vi "TLB Native Dynamic Events ver 0.26c.vi"() -> ()   [LabVIEW 2018] (continued)
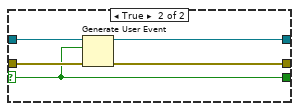
[diagram p2: hidden frame]
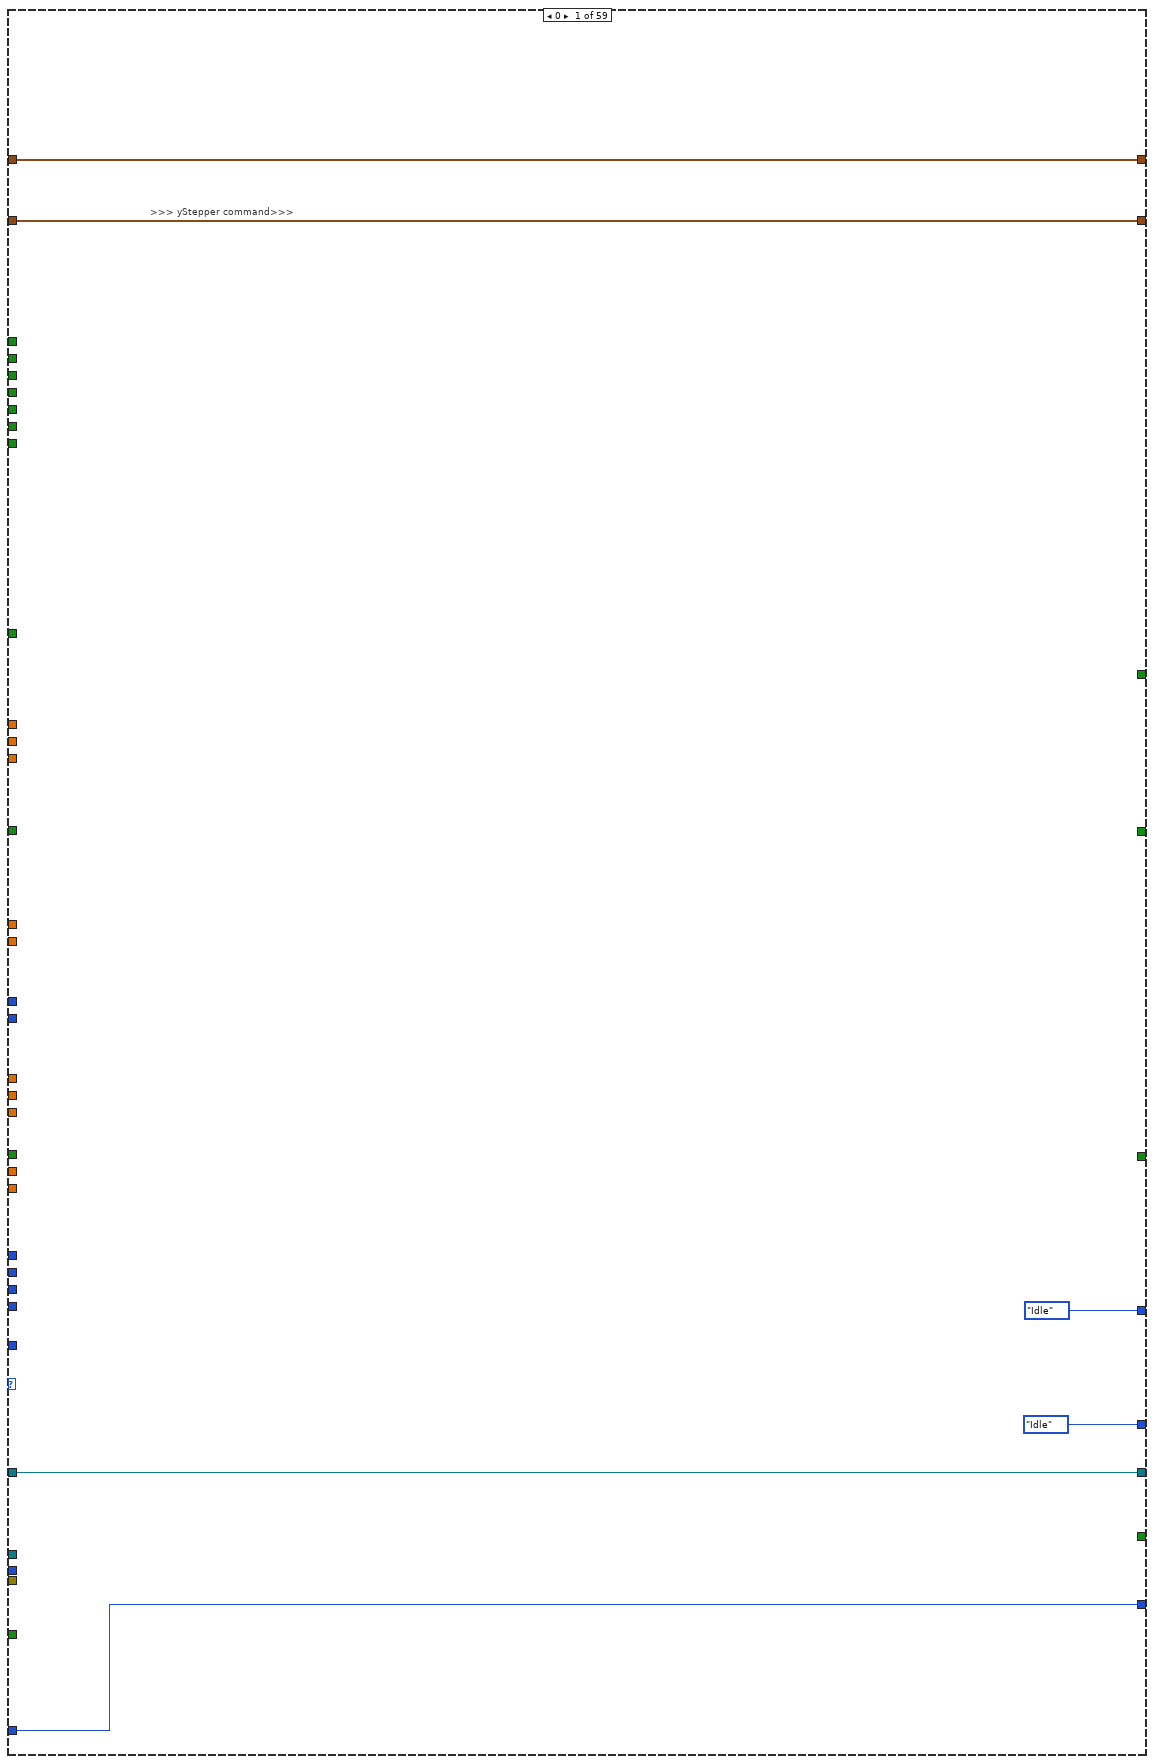
[diagram p5: hidden frame]
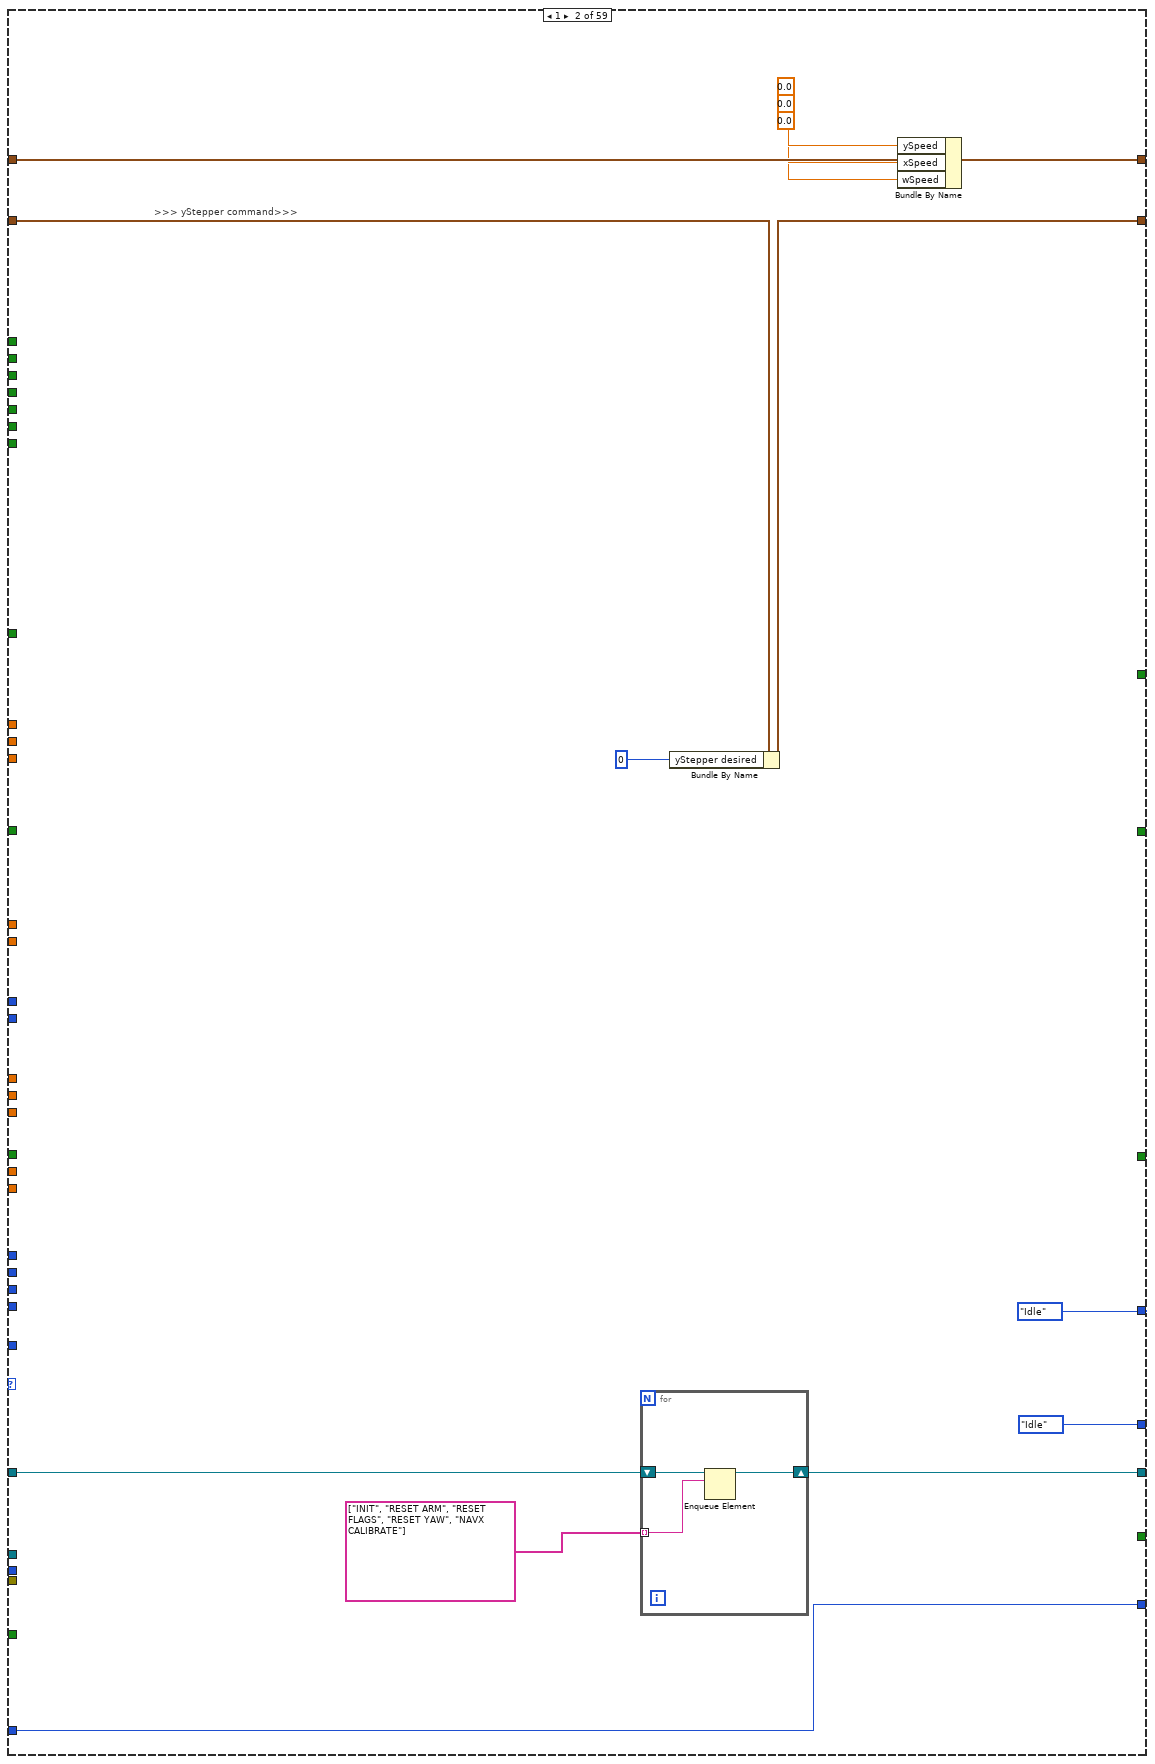
[diagram p6: hidden frame]
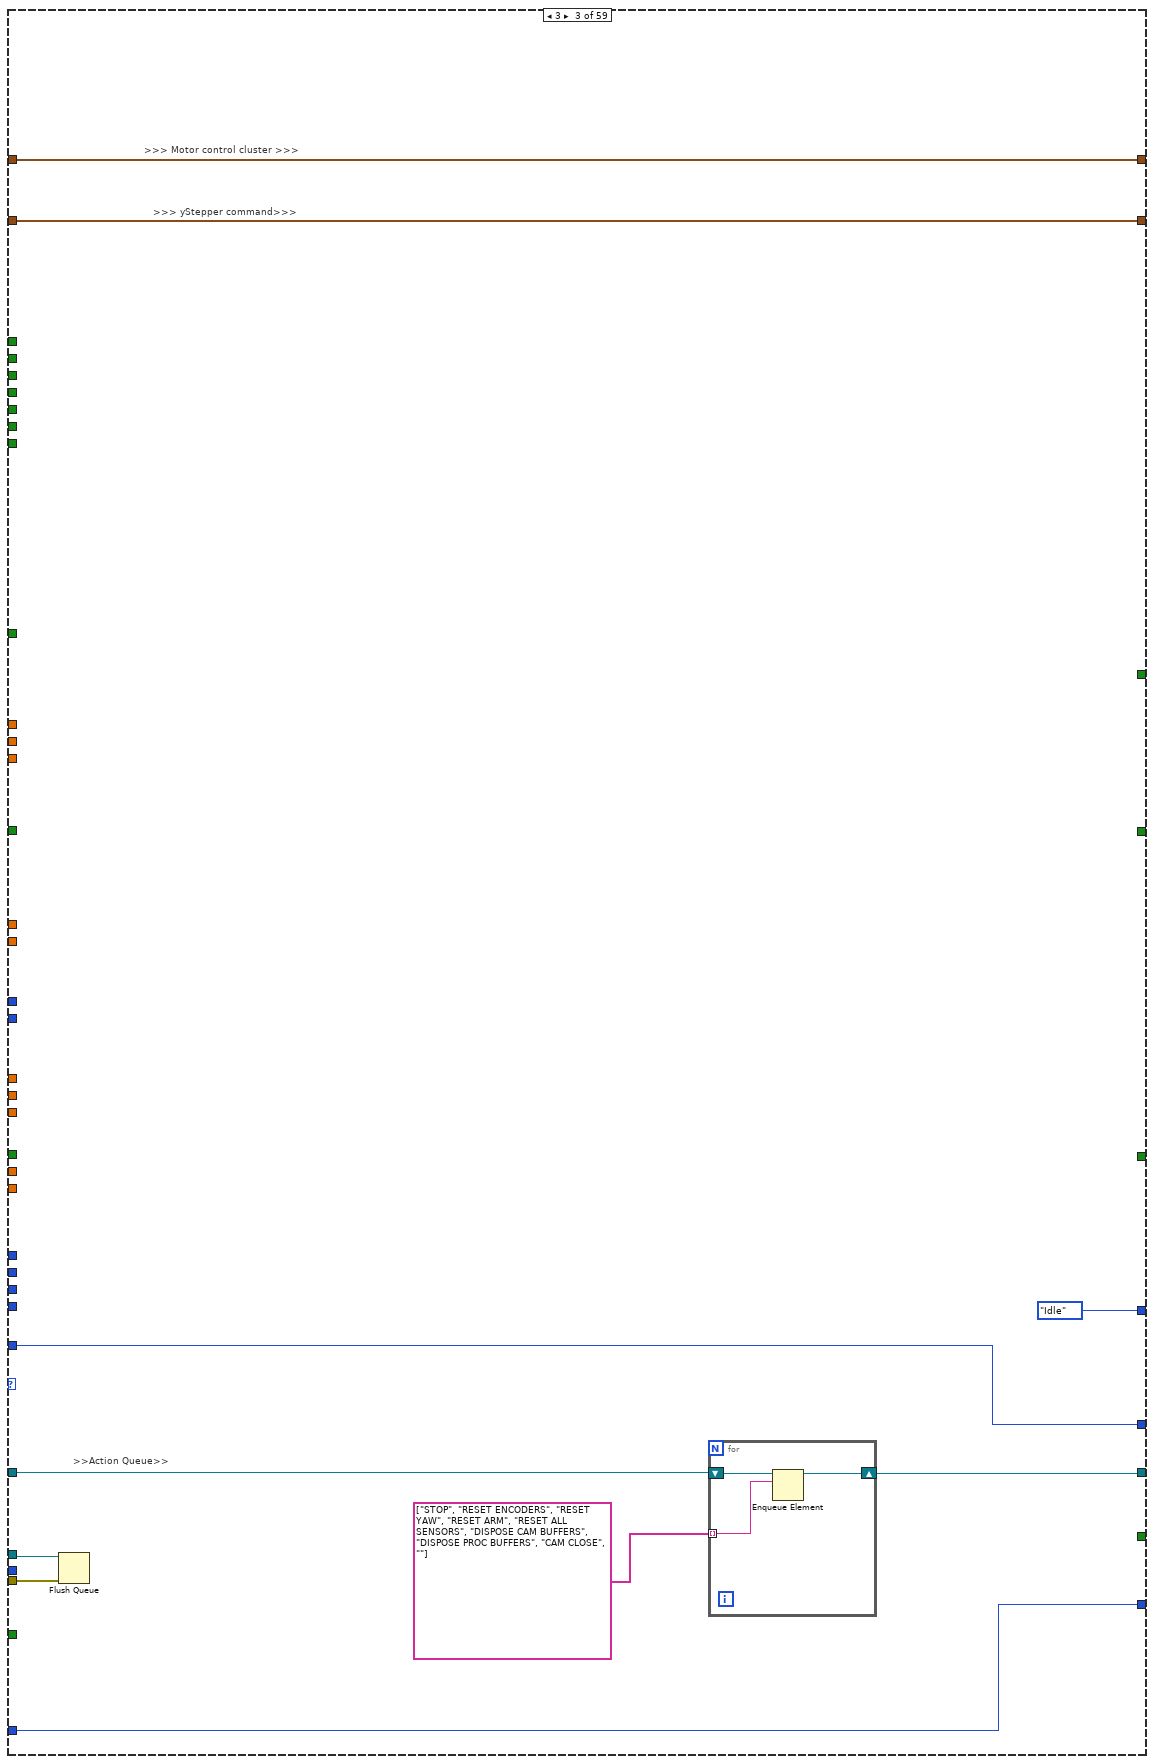
[diagram p7: hidden frame]
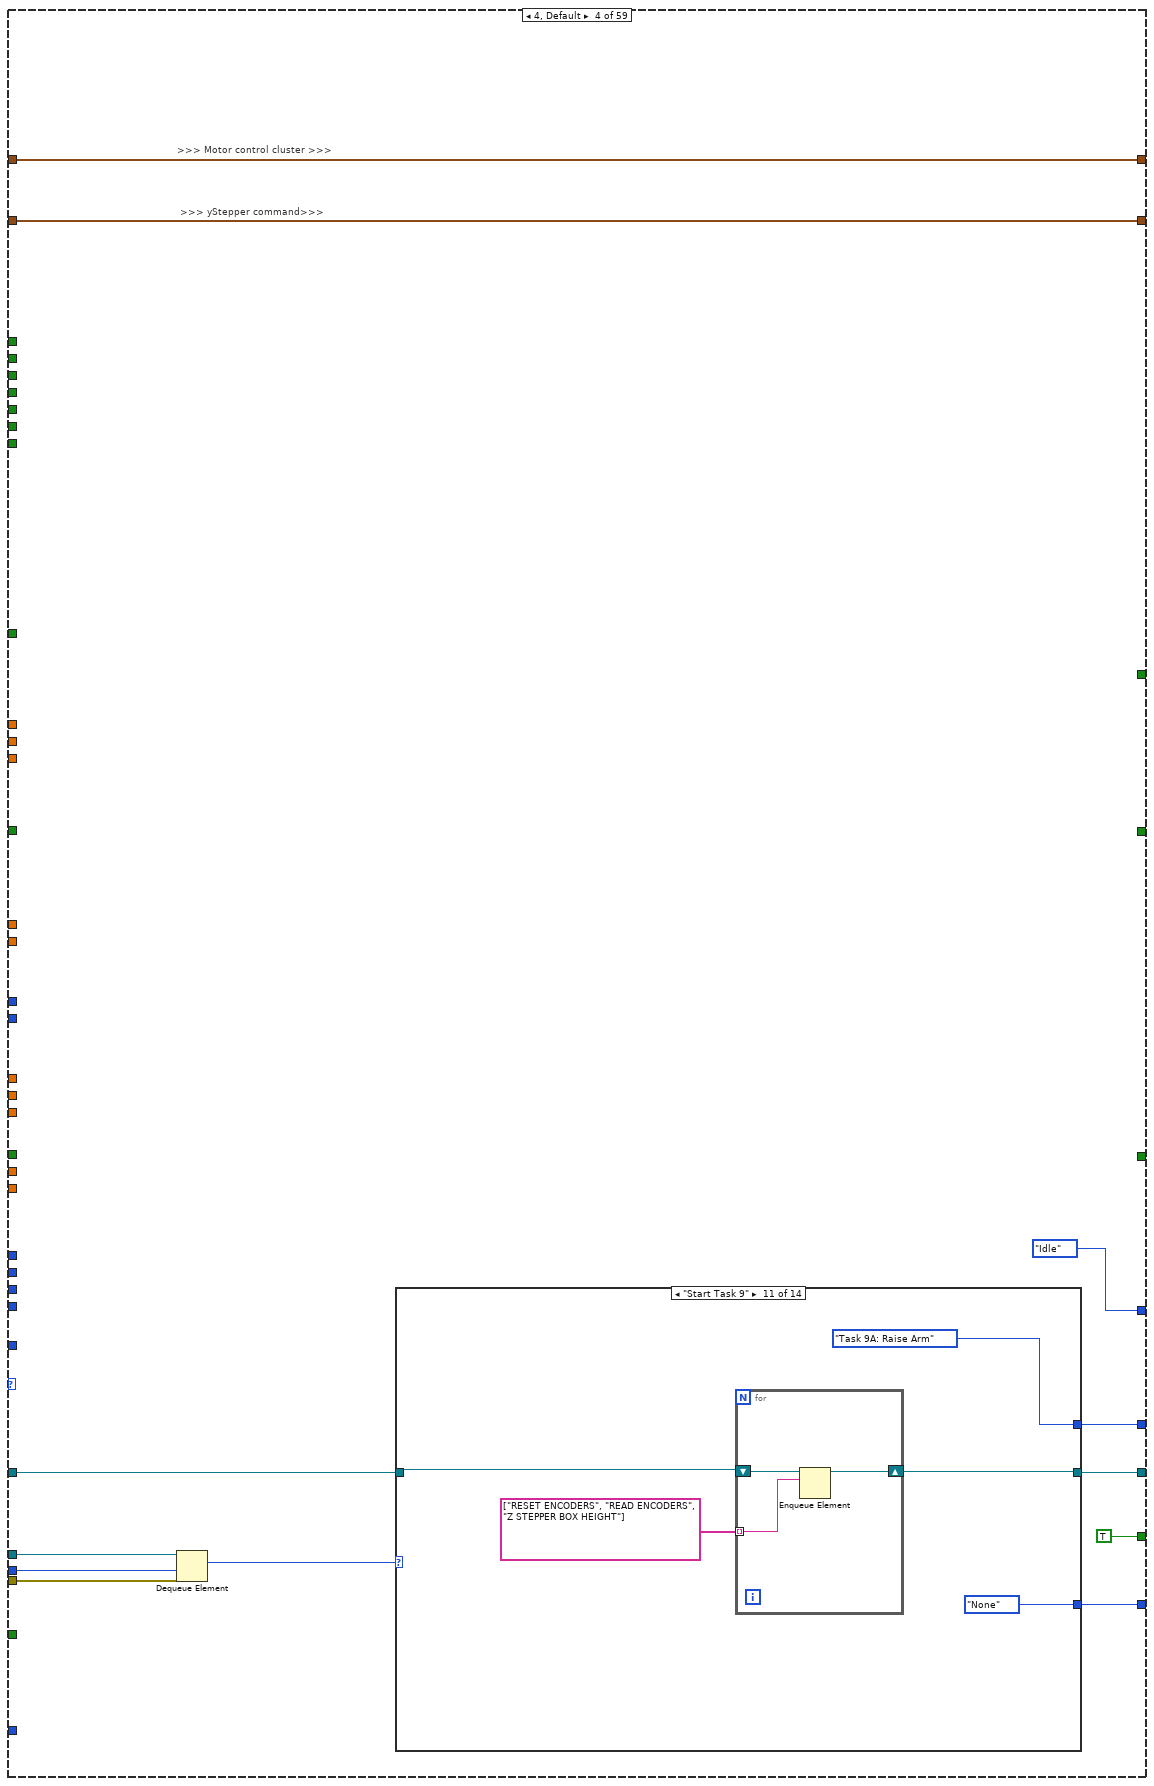
[diagram p8: hidden frame]
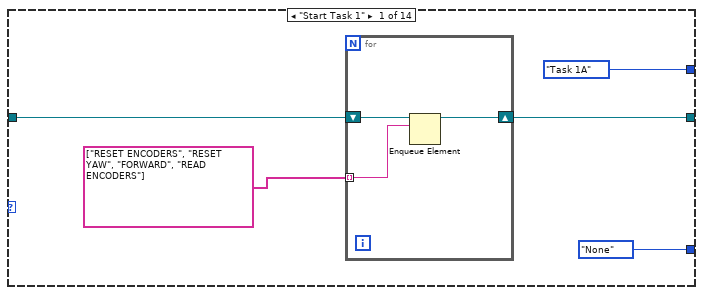
[diagram p9: hidden frame]
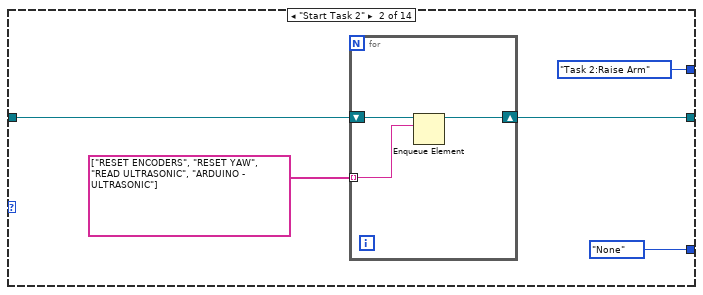
[diagram p10: hidden frame]
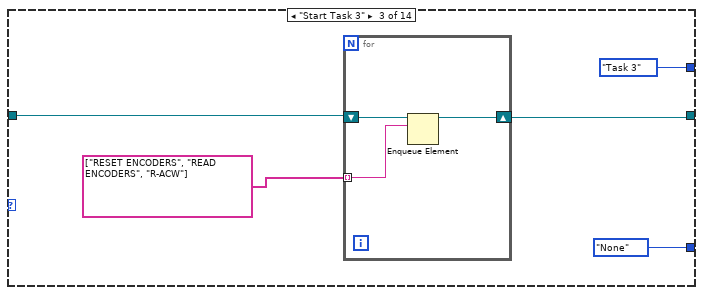
[diagram p11: hidden frame]
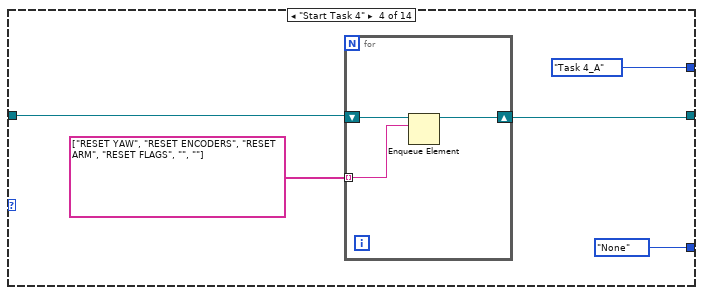
[diagram p12: hidden frame]
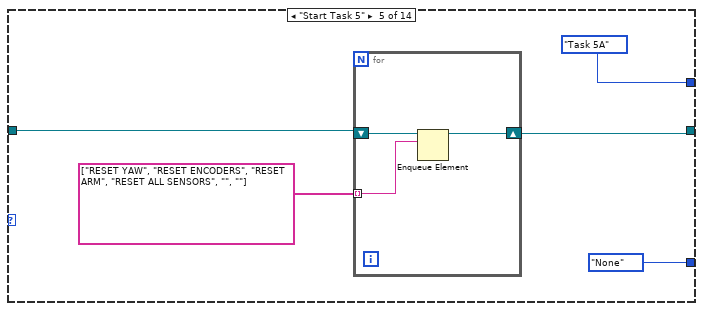
[diagram p13: hidden frame]
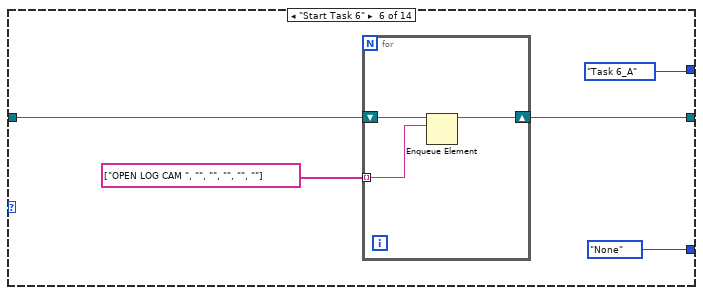
[diagram p14: hidden frame]
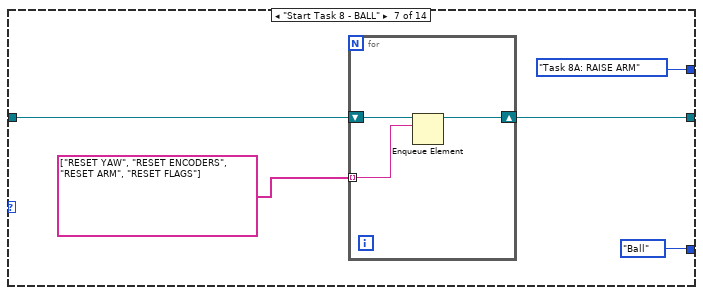
[diagram p15: hidden frame]
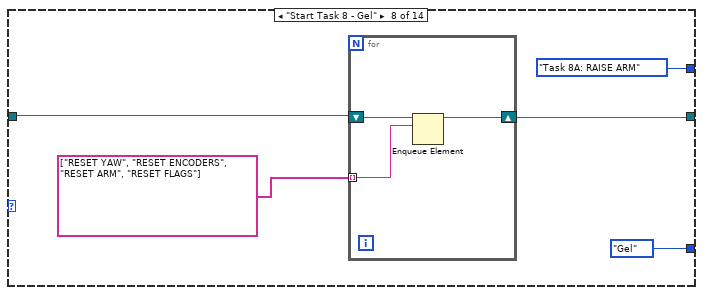
[diagram p16: hidden frame]
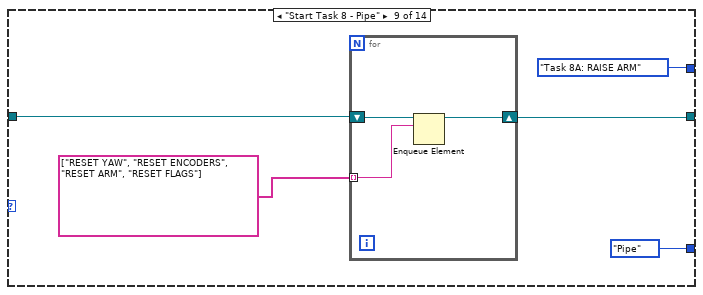
[diagram p17: hidden frame]
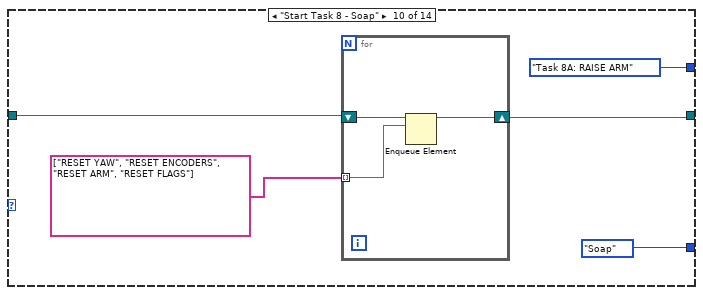
[diagram p18: hidden frame]
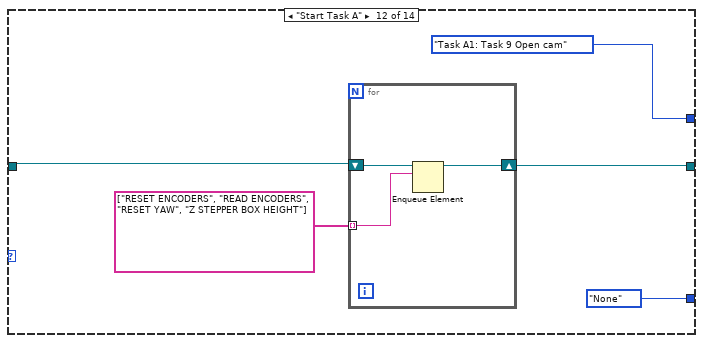
[diagram p19: hidden frame]
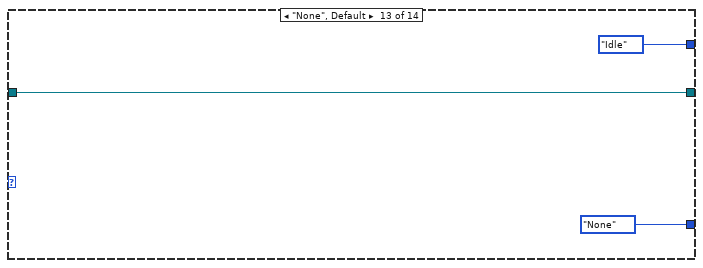
[diagram p20: hidden frame]
                  frame True {
                    n866 = for {
                      shift-right: [w2677] -> w2674
                      shift-left: w2675 -> [w2678]
                      tunnel: string[] ["STOP", "RESET ENCODERS", "RESET YAW", "OPEN LIFE CAM", "SET TIMER 2", "RESET FLAGS"] -> [w2676] mode=indexing
                      n867 = Enqueue Element(queue=w2678, element=w2676) -> (queue out=w2677:refnum<queue>)  [unwired: 2 in, 2 out]
                    }
                  }
                }
                n868 = Or(x=w2658, y=w2657) -> (x .or. y?=w2656:bool)
                n869 = Select(t=State_Type_Definitions,_for_0.26g_versions_and_later_2."True Stop" ("Enum"), s=w2657, f=State_Type_Definitions,_for_0.26d_versions_and_later."Task 9Q: SCAN IMAGE" ("Enum")) -> (s? t:f=w2659:u16)
                n870 = Select(t=w2659, s=w2656, f=State_Type_Definitions,_for_0.26d_versions_and_later."Task 9P: MOVE RIGHT" ("Enum")) -> (s? t:f=w2665:u16)
              }
              frame "Exit" {
                n871 = for {
                  shift-right: [w2685] -> w2682
                  shift-left: w2681 -> [w2686]
                  tunnel: string[] ["STOP", "RESET ENCODERS", "RESET YAW", "ARDUINO MODE 0"] -> [w2684] mode=indexing
                  n872 = Enqueue Element(queue=w2686, element=w2684) -> (queue out=w2685:refnum<queue>)  [unwired: 2 in, 2 out]
                }
              }
            }
          }
          frame 54 {
            # ">> Manual override >>"
            n873 = Dequeue Element(queue=w2695, timeout in ms (-1)=w2694, error in (no error)=w2693) -> (element=w2696:T10)  [unwired: 3 out]
            n874 = case shown="\"Start Task 1\", Default" w2696 {
              tunnel: [w2710 State_Type_Definitions,_for_0.26g_versions_and_later_2."True Stop" ("Enum")] -> w2688
              tunnel: [w2708 w2726] -> w2687
              tunnel: w2691 -> [w2707 w2723]
              tunnel: w2692 -> [w2701 _]
              tunnel: [State_Type_Definitions,_for_0.26g_versions_and_later_2."Idle" ("Enum") State_Type_Definitions,_for_0.26g_versions_and_later_2."Shutdown" ("Enum")] -> w2689
              tunnel: w2690 -> [w2700 _]
              frame "Start Task 1", Default {
                # ">> WIill proceed to part ii if not manual override >>"
                # ">>If ENABLE or Trigger is set to true>>"
                n875 = Or(x=w2700, y=w2701) -> (x .or. y?=w2702:bool)
                n876 = case shown="False" w2700 {
                  tunnel: [w2713 w2719] -> w2708
                  tunnel: w2707 -> [w2712 w2718]
                  frame False {
                    n877 = for {
                      shift-right: [w2715] -> w2713
                      shift-left: w2712 -> [w2716]
                      tunnel: string[] ["CAM ACQ", "START TIMER"] ("element") -> [w2714] mode=indexing
                      n878 = Enqueue Element(queue=w2716, element=w2714) -> (queue out=w2715:refnum<queue>)  [unwired: 2 in, 2 out]
                    }
                  }
                  frame True {
                    n879 = for {
                      shift-right: [w2721] -> w2719
                      shift-left: w2718 -> [w2722]
                      tunnel: string[] ["CLOSE CAM", "SET TIMER 5", "", "", "", ""] -> [w2720] mode=indexing
                      n880 = Enqueue Element(queue=w2722, element=w2720) -> (queue out=w2721:refnum<queue>)  [unwired: 2 in, 2 out]
                    }
                  }
                }
                n881 = Select(t=State_Type_Definitions,_for_0.26g_versions_and_later_2."True Stop" ("Enum"), s=w2701, f=State_Type_Definitions,_for_0.26g_versions_and_later_2."Task 9R: PROCESS COLOUR" ("Enum")) -> (s? t:f=w2704:T18)
                n882 = Select(t=w2704, s=w2702, f=State_Type_Definitions,_for_0.26d_versions_and_later."Task 9Q: SCAN IMAGE" ("Enum")) -> (s? t:f=w2710:u16)
              }
              frame "Exit" {
                n883 = for {
                  shift-right: [w2729] -> w2726
                  shift-left: w2723 -> [w2730]
                  tunnel: string[] ["STOP", "RESET ENCODERS", "RESET YAW", ""] -> [w2728] mode=indexing
                  n884 = Enqueue Element(queue=w2730, element=w2728) -> (queue out=w2729:refnum<queue>)  [unwired: 2 in, 2 out]
                }
              }
            }
          }
          frame 55 {
            # ">> Item Selection Bias >>"
            # ">>> Motor control cluster >>>"
            # ">>> yStepper command>>>"
            n885 = Dequeue Element(queue=w2736, timeout in ms (-1)=w2737, error in (no error)=w2738) -> (element=w2740:T10)  [unwired: 3 out]
            n886 = case shown="\"Start Task 1\", Default" w2740 {
              tunnel: w2734 -> [w2746 _]
              tunnel: [w2753 State_Type_Definitions,_for_0.26g_versions_and_later_2."True Stop" ("Enum")] -> w2732
              tunnel: w2739 -> [w2745 _]
              tunnel: w2735 -> [w2752 w2769]
              tunnel: [w2751 w2770] -> w2731
              tunnel: [State_Type_Definitions,_for_0.26g_versions_and_later_2."Idle" ("Enum") State_Type_Definitions,_for_0.26g_versions_and_later_2."Shutdown" ("Enum")] -> w2733
              frame "Start Task 1", Default {
                n887 = case shown="False" w2746 {
                  tunnel: w2752 -> [w2756 w2763]
                  tunnel: [w2757 w2762] -> w2751
                  frame False {
                    n888 = for {
                      tunnel: string[] ["START TIMER", "COLOUR PROCESSING", ""] ("element") -> [w2758] mode=indexing
                      shift-right: [w2760] -> w2757
                      shift-left: w2756 -> [w2759]
                      n889 = Enqueue Element(queue=w2759, element=w2758) -> (queue out=w2760:refnum<queue>)  [unwired: 2 in, 2 out]
                    }
                  }
                  frame True {
                    n890 = for {
                      shift-right: [w2765] -> w2762
                      shift-left: w2763 -> [w2766]
                      tunnel: string[] ["CLOSE CAM", "DISPOSE BUFFERS", "RESET ENCODERS", "RESET YAW", "RESET FLAGS", ""] -> [w2764] mode=indexing
                      n891 = Enqueue Element(queue=w2766, element=w2764) -> (queue out=w2765:refnum<queue>)  [unwired: 2 in, 2 out]
                    }
                  }
                }
                n892 = Or(x=w2746, y=w2745) -> (x .or. y?=w2744:bool)
                n893 = Select(t=State_Type_Definitions,_for_0.26g_versions_and_later_2."True Stop" ("Enum"), s=w2745, f=State_Type_Definitions,_for_0.26g_versions_and_later_2."True Stop" ("Enum")) -> (s? t:f=w2747:T18)
                n894 = Select(t=w2747, s=w2744, f=State_Type_Definitions,_for_0.26g_versions_and_later_2."Task 9R: PROCESS COLOUR" ("Enum")) -> (s? t:f=w2753:T18)
              }
              frame "Exit" {
                n895 = for {
                  shift-right: [w2773] -> w2770
                  shift-left: w2769 -> [w2774]
                  tunnel: string[] ["STOP", "RESET ENCODERS", "RESET YAW", "ARDUINO MODE 0"] -> [w2772] mode=indexing
                  n896 = Enqueue Element(queue=w2774, element=w2772) -> (queue out=w2773:refnum<queue>)  [unwired: 2 in, 2 out]
                }
              }
            }
          }
          frame 56 {
            # ">>> Motor control cluster >>>"
            # ">>> yStepper command>>>"
            # ">> Manual override >>"
            n897 = Dequeue Element(queue=w2786, timeout in ms (-1)=w2782, error in (no error)=w2785) -> (element=w2787:T10)  [unwired: 3 out]
            n898 = case shown="\"Start Task 1\", Default" w2787 {
              tunnel: [w2798 State_Type_Definitions,_for_0.26g_versions_and_later_2."True Stop" ("Enum")] -> w2780
              tunnel: [w2796 w2813] -> w2779
              tunnel: w2783 -> [w2795 _]
              tunnel: w2784 -> [w2789 _]
              tunnel: [State_Type_Definitions,_for_0.26g_versions_and_later_2."Idle" ("Enum") State_Type_Definitions,_for_0.26g_versions_and_later_2."Shutdown" ("Enum")] -> w2781
              tunnel: w2775 -> [w2788 _]
              frame "Start Task 1", Default {
                # ">> WIill proceed to part ii if not manual override >>"
                # ">>If ENABLE or Trigger is set to true>>"
                n899 = Or(x=w2788, y=w2789) -> (x .or. y?=w2790:bool)
                n900 = case shown="False" w2788 {
                  tunnel: [w2801 w2807] -> w2796
                  tunnel: w2795 -> [w2800 w2806]
                  frame False {
                    n901 = for {
                      shift-right: [w2803] -> w2801
                      shift-left: w2800 -> [w2804]
                      tunnel: string[] ["Task 9", ""] ("element") -> [w2802] mode=indexing
                      n902 = Enqueue Element(queue=w2804, element=w2802) -> (queue out=w2803:refnum<queue>)  [unwired: 2 in, 2 out]
                    }
                  }
                  frame True {
                    n903 = for {
                      shift-right: [w2809] -> w2807
                      shift-left: w2806 -> [w2810]
                      tunnel: string[] ["ARDUINO - ULTRASONIC", "READ NAVX", "RESET FLAGS", "", "", ""] -> [w2808] mode=indexing
                      n904 = Enqueue Element(queue=w2810, element=w2808) -> (queue out=w2809:refnum<queue>)  [unwired: 2 in, 2 out]
                    }
                  }
                }
                n905 = Select(t=State_Type_Definitions,_for_0.26g_versions_and_later_2."True Stop" ("Enum"), s=w2789, f=State_Type_Definitions,_for_0.26g_versions_and_later_2."True Stop" ("Enum")) -> (s? t:f=w2792:T18)
                n906 = Select(t=w2792, s=w2790, f=State_Type_Definitions,_for_0.26g_versions_and_later_2."Task A1: Task 9 Open cam" ("Enum")) -> (s? t:f=w2798:T18)
              }
              frame "Exit" {
                n907 = for {
                  shift-right: [w2816] -> w2813
                  shift-left: _ -> [w2817]
                  tunnel: string[] ["STOP", "RESET ENCODERS", "RESET YAW", ""] -> [w2815] mode=indexing
                  n908 = Enqueue Element(queue=w2817, element=w2815) -> (queue out=w2816:refnum<queue>)  [unwired: 2 in, 2 out]
                }
              }
            }
          }
          frame 57 {
            # ">>> Motor control cluster >>>"
            # ">>> yStepper command>>>"
            n909 = Dequeue Element(queue=w2831, timeout in ms (-1)=w2830, error in (no error)=w2829) -> (element=w2833:T10)  [unwired: 3 out]
            n910 = In Range and Coerce(upper limit=65.0, x=w2823, lower limit=58.0) -> (In Range?=w2820:bool)  [unwired: 1 out]
            n911 = case shown="\"Start Task 1\", Default" w2833 {
              tunnel: w2824 -> [w2836 _]
              tunnel: [w2844 State_Type_Definitions,_for_0.26g_versions_and_later_2."True Stop" ("Enum")] -> w2826
              tunnel: w2832 -> [w2842 w2860]
              tunnel: [w2841 w2859] -> w2825
              tunnel: [State_Type_Definitions,_for_0.26g_versions_and_later_2."Idle" ("Enum") State_Type_Definitions,_for_0.26g_versions_and_later_2."Shutdown" ("Enum")] -> w2827
              tunnel: w2820 -> [w2834 _]
              frame "Start Task 1", Default {
                n912 = Or(x=w2834, y=w2836) -> (x .or. y?=w2835:bool)
                n913 = case shown="True" w2834 {
                  tunnel: w2842 -> [w2847 w2853]
                  tunnel: [w2846 w2851] -> w2841
                  frame False {
                    n914 = for {
                      shift-right: [w2849] -> w2846
                      shift-left: w2847 -> [w2850]
                      tunnel: string[] ["READ NAVX", "R-CW", "READ ULTRASONIC"] ("element") -> [w2848] mode=indexing
                      n915 = Enqueue Element(queue=w2850, element=w2848) -> (queue out=w2849:refnum<queue>)  [unwired: 2 in, 2 out]
                    }
                  }
                  frame True {
                    n916 = for {
                      shift-right: [w2855] -> w2851
                      shift-left: w2853 -> [w2856]
                      tunnel: string[] ["STOP", "RESET ENCODERS", "RESET YAW", "READ IR", "ARDUINO - ULTRASONIC"] -> [w2854] mode=indexing
                      n917 = Enqueue Element(queue=w2856, element=w2854) -> (queue out=w2855:refnum<queue>)  [unwired: 2 in, 2 out]
                    }
                  }
                }
                n918 = Select(t=State_Type_Definitions,_for_0.26g_versions_and_later_2."True Stop" ("Enum"), s=w2836, f=State_Type_Definitions,_for_0.26g_versions_and_later_2."Task A3: Task 9 Set Timer") -> (s? t:f=w2838:T18)
                n919 = Select(t=w2838, s=w2835, f=State_Type_Definitions,_for_0.26g_versions_and_later_2."Task A2: Task 9 Move Arm" ("Enum")) -> (s? t:f=w2844:T18)
              }
              frame "Exit" {
                n920 = for {
                  shift-right: [w2863] -> w2859
                  shift-left: w2860 -> [w2864]
                  tunnel: string[] ["STOP", "RESET ENCODERS", "RESET YAW", ""] -> [w2862] mode=indexing
                  n921 = Enqueue Element(queue=w2864, element=w2862) -> (queue out=w2863:refnum<queue>)  [unwired: 2 in, 2 out]
                }
              }
            }
          }
          frame 58 {
            (unwired) 50.0 ("y")
            (unwired) 15.0 ("y")
            # ">> Item Selection Bias >>"
            # ">> Wall detected >>"
            # ">> Manual override >>"
            # ">>> Motor control cluster >>>"
            # ">>Table or wall detectected>>"
            # ">>Action Queue>>"
            # ">>> yStepper command>>>"
            n922 = Dequeue Element(queue=w2880, timeout in ms (-1)=w2879, error in (no error)=w2878) -> (element=w2881:T10)  [unwired: 3 out]
            n923 = Less?(x=w2867, y=100.0) -> (x < y?=w2868:bool)
            n924 = Not Equal To 0?(x=w2867) -> (x != 0?=w2866:bool)
            n925 = And(x=w2866, y=w2868) -> (x .and. y?=w2865:bool)
            n926 = case shown="\"Start Task 1\", Default" w2881 {
              tunnel: w2876 -> [w2882 _]
              tunnel: [w2892 State_Type_Definitions,_for_0.26g_versions_and_later_2."True Stop" ("Enum")] -> w2873
              tunnel: w2877 -> [w2890 w2908]
              tunnel: [w2889 w2907] -> w2872
              tunnel: [State_Type_Definitions,_for_0.26g_versions_and_later_2."Idle" ("Enum") State_Type_Definitions,_for_0.26g_versions_and_later_2."Shutdown" ("Enum")] -> w2875
              tunnel: w2865 -> [w2883 _]
              frame "Start Task 1", Default {
                n927 = Or(x=w2882, y=w2883) -> (x .or. y?=w2884:bool)
                n928 = case shown="False" w2883 {
                  tunnel: w2890 -> [w2895 w2901]
                  tunnel: [w2894 w2899] -> w2889
                  frame False {
                    n929 = for {
                      shift-right: [w2897] -> w2894
                      shift-left: w2895 -> [w2898]
                      tunnel: string[] ["READ IR", "FORWARD - IR ASSIST", "READ ULTRASONIC"] ("element") -> [w2896] mode=indexing
                      n930 = Enqueue Element(queue=w2898, element=w2896) -> (queue out=w2897:refnum<queue>)  [unwired: 2 in, 2 out]
                    }
                  }
                  frame True {
                    n931 = for {
                      shift-right: [w2903] -> w2899
                      shift-left: w2901 -> [w2904]
                      tunnel: string[] ["STOP", "RESET ENCODERS", "RESET YAW", ""] -> [w2902] mode=indexing
                      n932 = Enqueue Element(queue=w2904, element=w2902) -> (queue out=w2903:refnum<queue>)  [unwired: 2 in, 2 out]
                    }
                  }
                }
                n933 = Select(t=State_Type_Definitions,_for_0.26g_versions_and_later_2."True Stop" ("Enum"), s=w2882, f=State_Type_Definitions,_for_0.26g_versions_and_later_2."Task A4: Tasl 9 Capture images") -> (s? t:f=w2886:T18)
                n934 = Select(t=w2886, s=w2884, f=State_Type_Definitions,_for_0.26g_versions_and_later_2."Task A3: Task 9 Set Timer" ("Enum")) -> (s? t:f=w2892:T18)
              }
              frame "Exit" {
                n935 = for {
                  shift-right: [w2911] -> w2907
                  shift-left: w2908 -> [w2912]
                  tunnel: string[] ["STOP", "RESET ENCODERS", "RESET YAW", ""] -> [w2910] mode=indexing
                  n936 = Enqueue Element(queue=w2912, element=w2910) -> (queue out=w2911:refnum<queue>)  [unwired: 2 in, 2 out]
                }
              }
            }
          }
          frame 59 {
            # ">>> Motor control cluster >>>"
            # ">>> yStepper command>>>"
            # ">> Item Selection Bias >>"
            n937 = Less?(x=w2916, y=-40.0) -> (x < y?=w2914:bool)
            n938 = Dequeue Element(queue=w2922, timeout in ms (-1)=w2921, error in (no error)=w2920) -> (element=w2924:T10)  [unwired: 3 out]
            n939 = case shown="\"Start Task 1\", Default" w2924 {
              tunnel: w2914 -> [w2930 _]
              tunnel: [w2937 State_Type_Definitions,_for_0.26g_versions_and_later_2."True Stop" ("Enum")] -> w2918
              tunnel: w2919 -> [w2929 _]
              tunnel: w2923 -> [w2936 w2953]
              tunnel: [w2935 w2954] -> w2913
              tunnel: [State_Type_Definitions,_for_0.26g_versions_and_later_2."Idle" ("Enum") State_Type_Definitions,_for_0.26g_versions_and_later_2."Shutdown" ("Enum")] -> w2917
              frame "Start Task 1", Default {
                n940 = case shown="True" w2930 {
                  tunnel: w2936 -> [w2940 w2947]
                  tunnel: [w2941 w2946] -> w2935
                  frame False {
                    n941 = for {
                      tunnel: string[] ["READ ENCODERS", "R-CW"] ("element") -> [w2942] mode=indexing
                      shift-right: [w2944] -> w2941
                      shift-left: w2940 -> [w2943]
                      n942 = Enqueue Element(queue=w2943, element=w2942) -> (queue out=w2944:refnum<queue>)  [unwired: 2 in, 2 out]
                    }
                  }
                  frame True {
                    n943 = for {
                      shift-right: [w2949] -> w2946
                      shift-left: w2947 -> [w2950]
                      tunnel: string[] ["STOP", "RESET ENCODERS", "RESET FLAGS", "RESET YAW", "READ IR", ""] -> [w2948] mode=indexing
                      n944 = Enqueue Element(queue=w2950, element=w2948) -> (queue out=w2949:refnum<queue>)  [unwired: 2 in, 2 out]
                    }
                  }
                }
                n945 = Or(x=w2930, y=w2929) -> (x .or. y?=w2928:bool)
                n946 = Select(t=State_Type_Definitions,_for_0.26g_versions_and_later_2."True Stop" ("Enum"), s=w2929, f=State_Type_Definitions,_for_0.26g_versions_and_later_2."Task A3: Task 9 Set Timer" ("Enum")) -> (s? t:f=w2931:T18)
                n947 = Select(t=w2931, s=w2928, f=State_Type_Definitions,_for_0.26g_versions_and_later_2."Task A4: Tasl 9 Capture images" ("Enum")) -> (s? t:f=w2937:T18)
              }
              frame "Exit" {
                n948 = for {
                  shift-right: [w2957] -> w2954
                  shift-left: w2953 -> [w2958]
                  tunnel: string[] ["STOP", "RESET ENCODERS", "RESET YAW", "ARDUINO MODE 0"] -> [w2956] mode=indexing
                  n949 = Enqueue Element(queue=w2958, element=w2956) -> (queue out=w2957:refnum<queue>)  [unwired: 2 in, 2 out]
                }
              }
            }
          }
        }
        "Object Detection" <- w320
        "Ultrasonic sensors" <- w343
        "Encoder values" <- w332
        "Stepper position values" <- w316
        "NAVX Values" <- w314
        "IR Sensors" <- w306
        "Line sensors" <- w301
        "Time cluster" <- w312
        "Box Colour Detection" <- w294
      }
    }
    "Object recognition mode" <- w220
    "Front Ultrasonic obstruct" <- w217
    "Front IR obstruct" <- w216
    "Table IR obstruct" <- w215
    n950 = local write "Green LED"(w230) -> ()
  }
  n951 = while {
    stop <- w3838 stop-if-true
    n952 = call "MOTOR CONTROL WITH PID AE.vi"("AE Mode"=MOTOR_CONTROL_WITH_PID_AE_DATA_MODE_TYPE_DEF."Read from AE") -> ("Speed & distance"=→"Speed & distance":T15)  [unwired: 3 in]
    n953 = call "FGV Stop.vi"("Init/Read/Write State"=States_for_Action_Engine."Read") -> ("Output node"=w3838:bool)  [unwired: 2 in, 1 out]
    n954 = Wait (ms)(milliseconds to wait=u32 5) -> ()  [unwired: 1 out]
  }
  n955 = call <vilib>:"DIO Close.vi"("error in (no error)"=w23, "DIO Info In"=w26) -> ()  [unwired: 9 in, 1 out]
  n956 = call <vilib>:"DIO Close.vi"("error in (no error)"=w33, "DIO Info In"=w35) -> ()  [unwired: 9 in, 1 out]
  n957 = call <vilib>:"NavX Close.vi"("error in (no error)"=w10, "NavX Info In"=w9) -> ()  [unwired: 9 in, 1 out]
  n958 = call <vilib>:"DIO Close.vi"("error in (no error)"=w28, "DIO Info In"=w30) -> ()  [unwired: 9 in, 1 out]
  n959 = call <vilib>:"DIO Close.vi"("error in (no error)"=w17, "DIO Info In"=w18) -> ()  [unwired: 9 in, 1 out]
  n960 = call <vilib>:"DIO Close.vi"("error in (no error)"=w12, "DIO Info In"=w13) -> ()  [unwired: 9 in, 1 out]
  n961 = Merge Errors "Merge Errors"(w63, w62) -> (w45:errorcluster)
  n962 = Merge Errors(w49, w45) -> (w44:errorcluster)
  n963 = Destroy User Event(user event=w67, error in=w44) -> ()  [unwired: 1 out]
  n964 = Release Queue(queue=w40, error in (no error)=w44) -> (error out=→"Queue Errors":errorcluster)  [unwired: 1 in, 2 out]
  n965 = Release Queue(queue=w57, error in (no error)=w44) -> ()  [unwired: 1 in, 3 out]
  n966 = Destroy User Event(user event=w66, error in=w44) -> ()  [unwired: 1 out]
  n967 = Unregister For Events(event registration refnum=w58, error in=w44) -> ()  [unwired: 1 out]
